vi "ScanDelay_FTIR_PointSpectroscopy.vi"() -> ()   [LabVIEW 2022 SP3] (continued)
  in  "BB-reference spectrum":bool
  in  "Acquire only\nBB 100% curve":bool
  in  "Toggle pause (ms)":dbl=1000.0
  out "BB-referenced spectrum (phase)":T1(graph)
  out "BB-referenced spectrum (amplitude)":T2(graph)
  out "Reference BB spectra":dbl[][](array[numeric])
  out "Reference spectra":dbl[][](array[numeric])
  out "Latest alpha cmd":string="@mir setpump 50.0"
  in  "Replicate\nalpha on\naccumulation":bool=TRUE
  out "# Accumulated":i32=21
  in  "Accumulate to #":i32=21
  in  "Cancel\nacquisition":bool
  out "Toggle position":i32=2
  out "Spectrum stored":bool=TRUE
  out "Reference stored":bool=TRUE
  out "Normalized spectrum (phase)":T1(graph)
  out "Normalized spectrum (amplitude)":T1(graph)
  in  "Store as reference":bool
  out "Python alpha rep path":path=path "C:/Users/mnopl/Desktop/software/mnOPSuite/PRISM/python/alpha.py"
  out "Activity status":string="Awaiting command"
  out "Acquisition status":string="Ready to acquire spectrum"
  in  "Path to save spectrum":path=path "D:/Dropbox/Data/Park-SNOM/2022.07.19 - Liam - Strained STO/11_30 Measurements/Spectra/S2_AuRef12_9.txt"
  in  "Load reference":bool
  in  "Path to load reference":path=path "D:/Dropbox/Data/Park-SNOM/2022.07.19 - Liam - Strained STO/12_7 Measurements/STO_undeformed_S2.txt"
  in  "Path to load spectrum":path=path "D:/Dropbox/Data/Park-SNOM/2022.07.19 - Liam - Strained STO/12_7 Measurements/STO_undeformed_S2.txt"
  in  "Apply spectral\nenvelope":bool=TRUE
  out "Binned interferogram":cluster{"X":dbl, "Y":dbl}[](graph)
  out "Sample BB Spectra":dbl[][](array[numeric])
  out "Sample Spectra":dbl[][](array[numeric])
  out "Python error: spectrum acquisition":errorcluster
  out "Python scandelay path":path=path "C:/Users/mnopl/Desktop/software/mnOPSuite/PRISM/python/scandelay_FTIR.py"
  in  "Time per\nacquisition (s)":dbl=0.18
  in  "Sampling rate":dbl=250000.0
  in  "Delay calibratior\nfactor (ps/V)":dbl=-2.432 format="%_6g"
  in  "Cyc. / intfg.\n(sample)":i32=150
  out "Accumulated spectrum (amplitude)":T3(graph)
  out "Acquisition cycle":dbl[][](graph)
  out "% averaged":dbl=100.0
  in  "Halt program":bool=TRUE
  out "Python error: activity loop":errorcluster
  in  "Load spectrum":bool
  in  "Save spectrum":bool
  in  "Normalize spectrum":bool
  in  "Acquire spectrum":bool
  # "ai6 (7ps): -2 to -5"
  # "ai2 (7ps): -12 to -15"
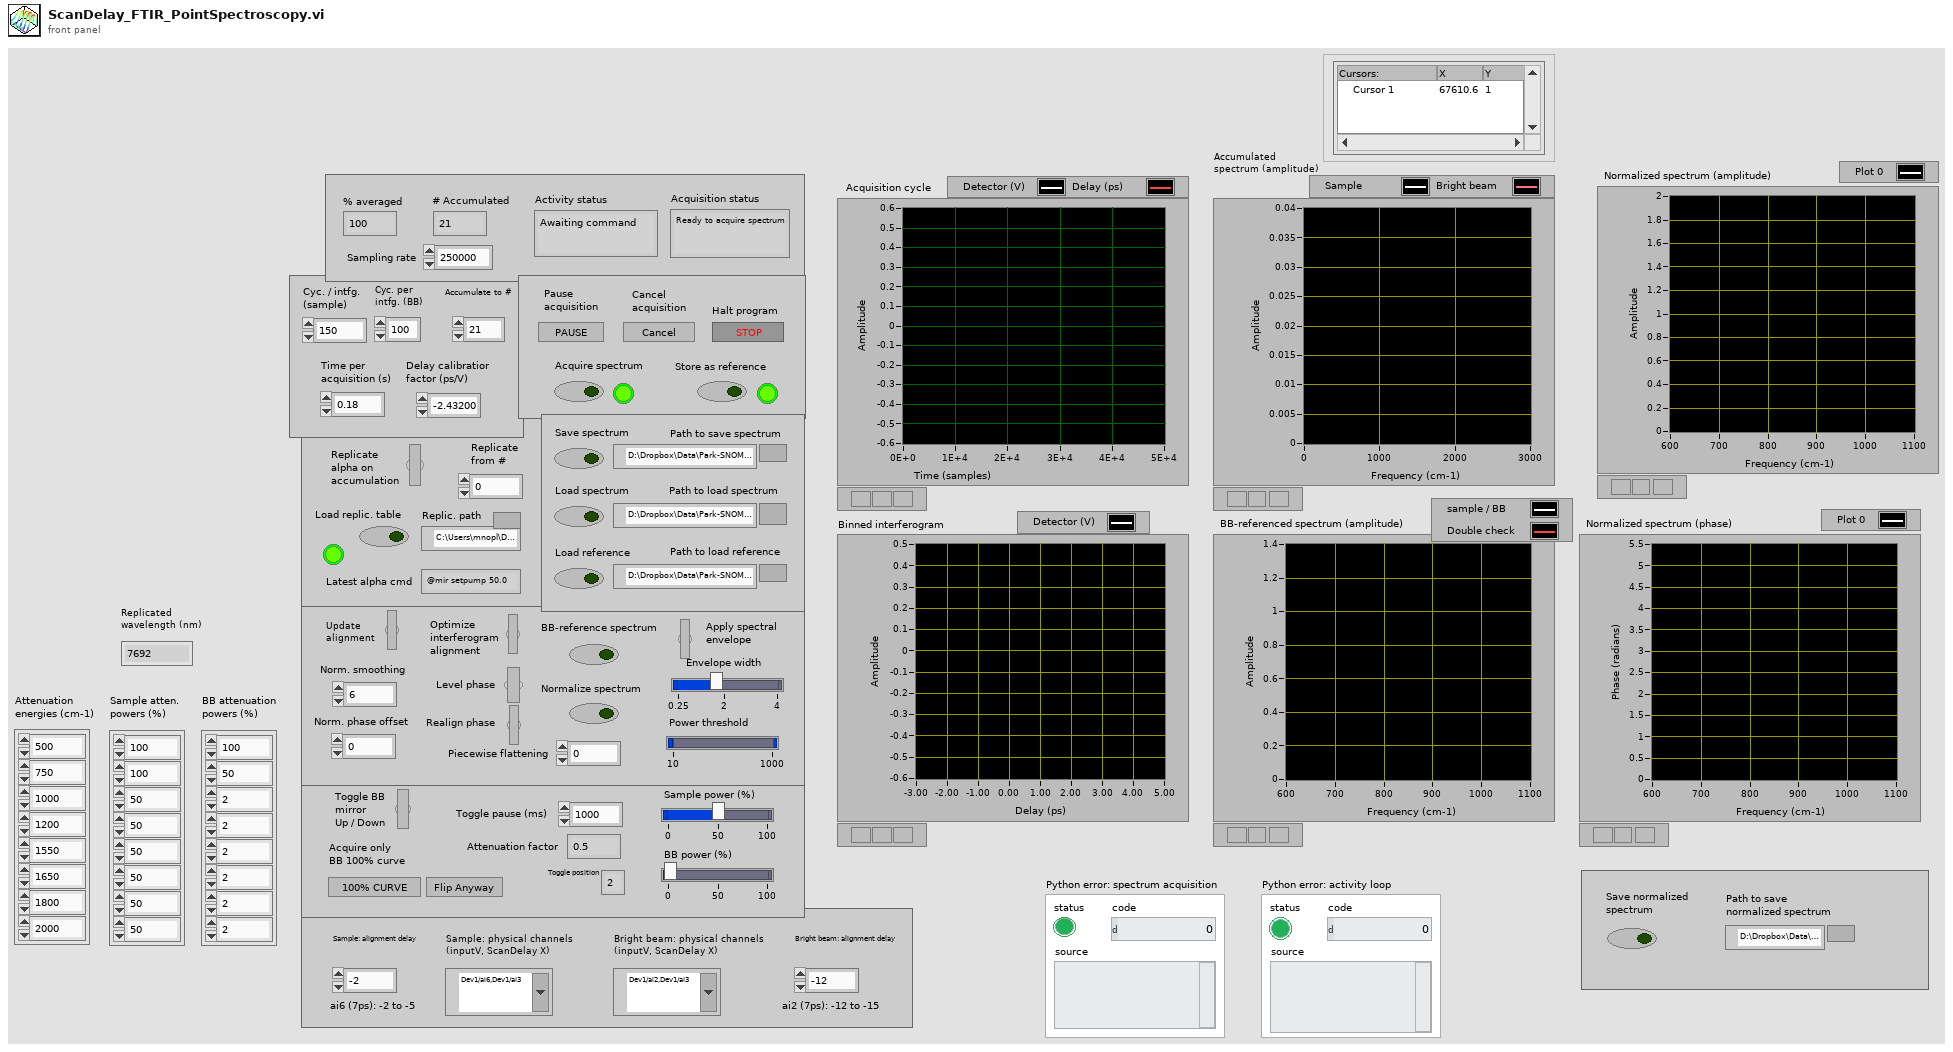
[diagram p1: front panel]
types:
  T1 = cluster{"Output spectrum":dbl[], "Output spectrum":dbl[]}
  T2 = cluster{"Sample Spectra":dbl[], "Sample Spectra":dbl[]}
  T3 = cluster{"Output spectrum":dbl[], "Output spectrum":dbl[]}[]
  T4 = typedef "Control_scanDelayWorkflow.ctl" = enum16{"Hyperspectrum at point", "Sit Idle", "Initialize", "Unpack hyperspectrum", "Slice hyperspectrum", "Linecut norm. at position", "Linecut norm. at frequency", "Next Point", "Load replicator table", "Flip BB", "Load Spectrum", "Store reference", "Save Spectrum", "Load reference", "Check Reference", "Check Spectrum", "Heal linescan", "BB reference spectrum", "BB reference linescan", "Normalize Spectrum", "Normalize Linescan", "Save normalized spectrum", "Save Linescan", "Load Linescan", "Done"}
  T5 = typedef "imagedata.ctl" = cluster{"image type":i32, "image depth":i32, "image":u8[], "mask":u8[], "colors":u32[], "Rectangle":cluster{"left":i16, "top":i16, "right":i16, "bottom":i16}}
  T6 = typedef "Control_GetSpectrum_BBnorm_AttenuateBB.ctl" = enum16{"Initialize", "Replicate alpha", "Flip in BB", "Attenuate alpha", "Get Spectrum", "Accumulate BB spectrum", "Flip out BB", "Accumulate sample spectrum", "Assess accumulation", "Finalize", "Done"}
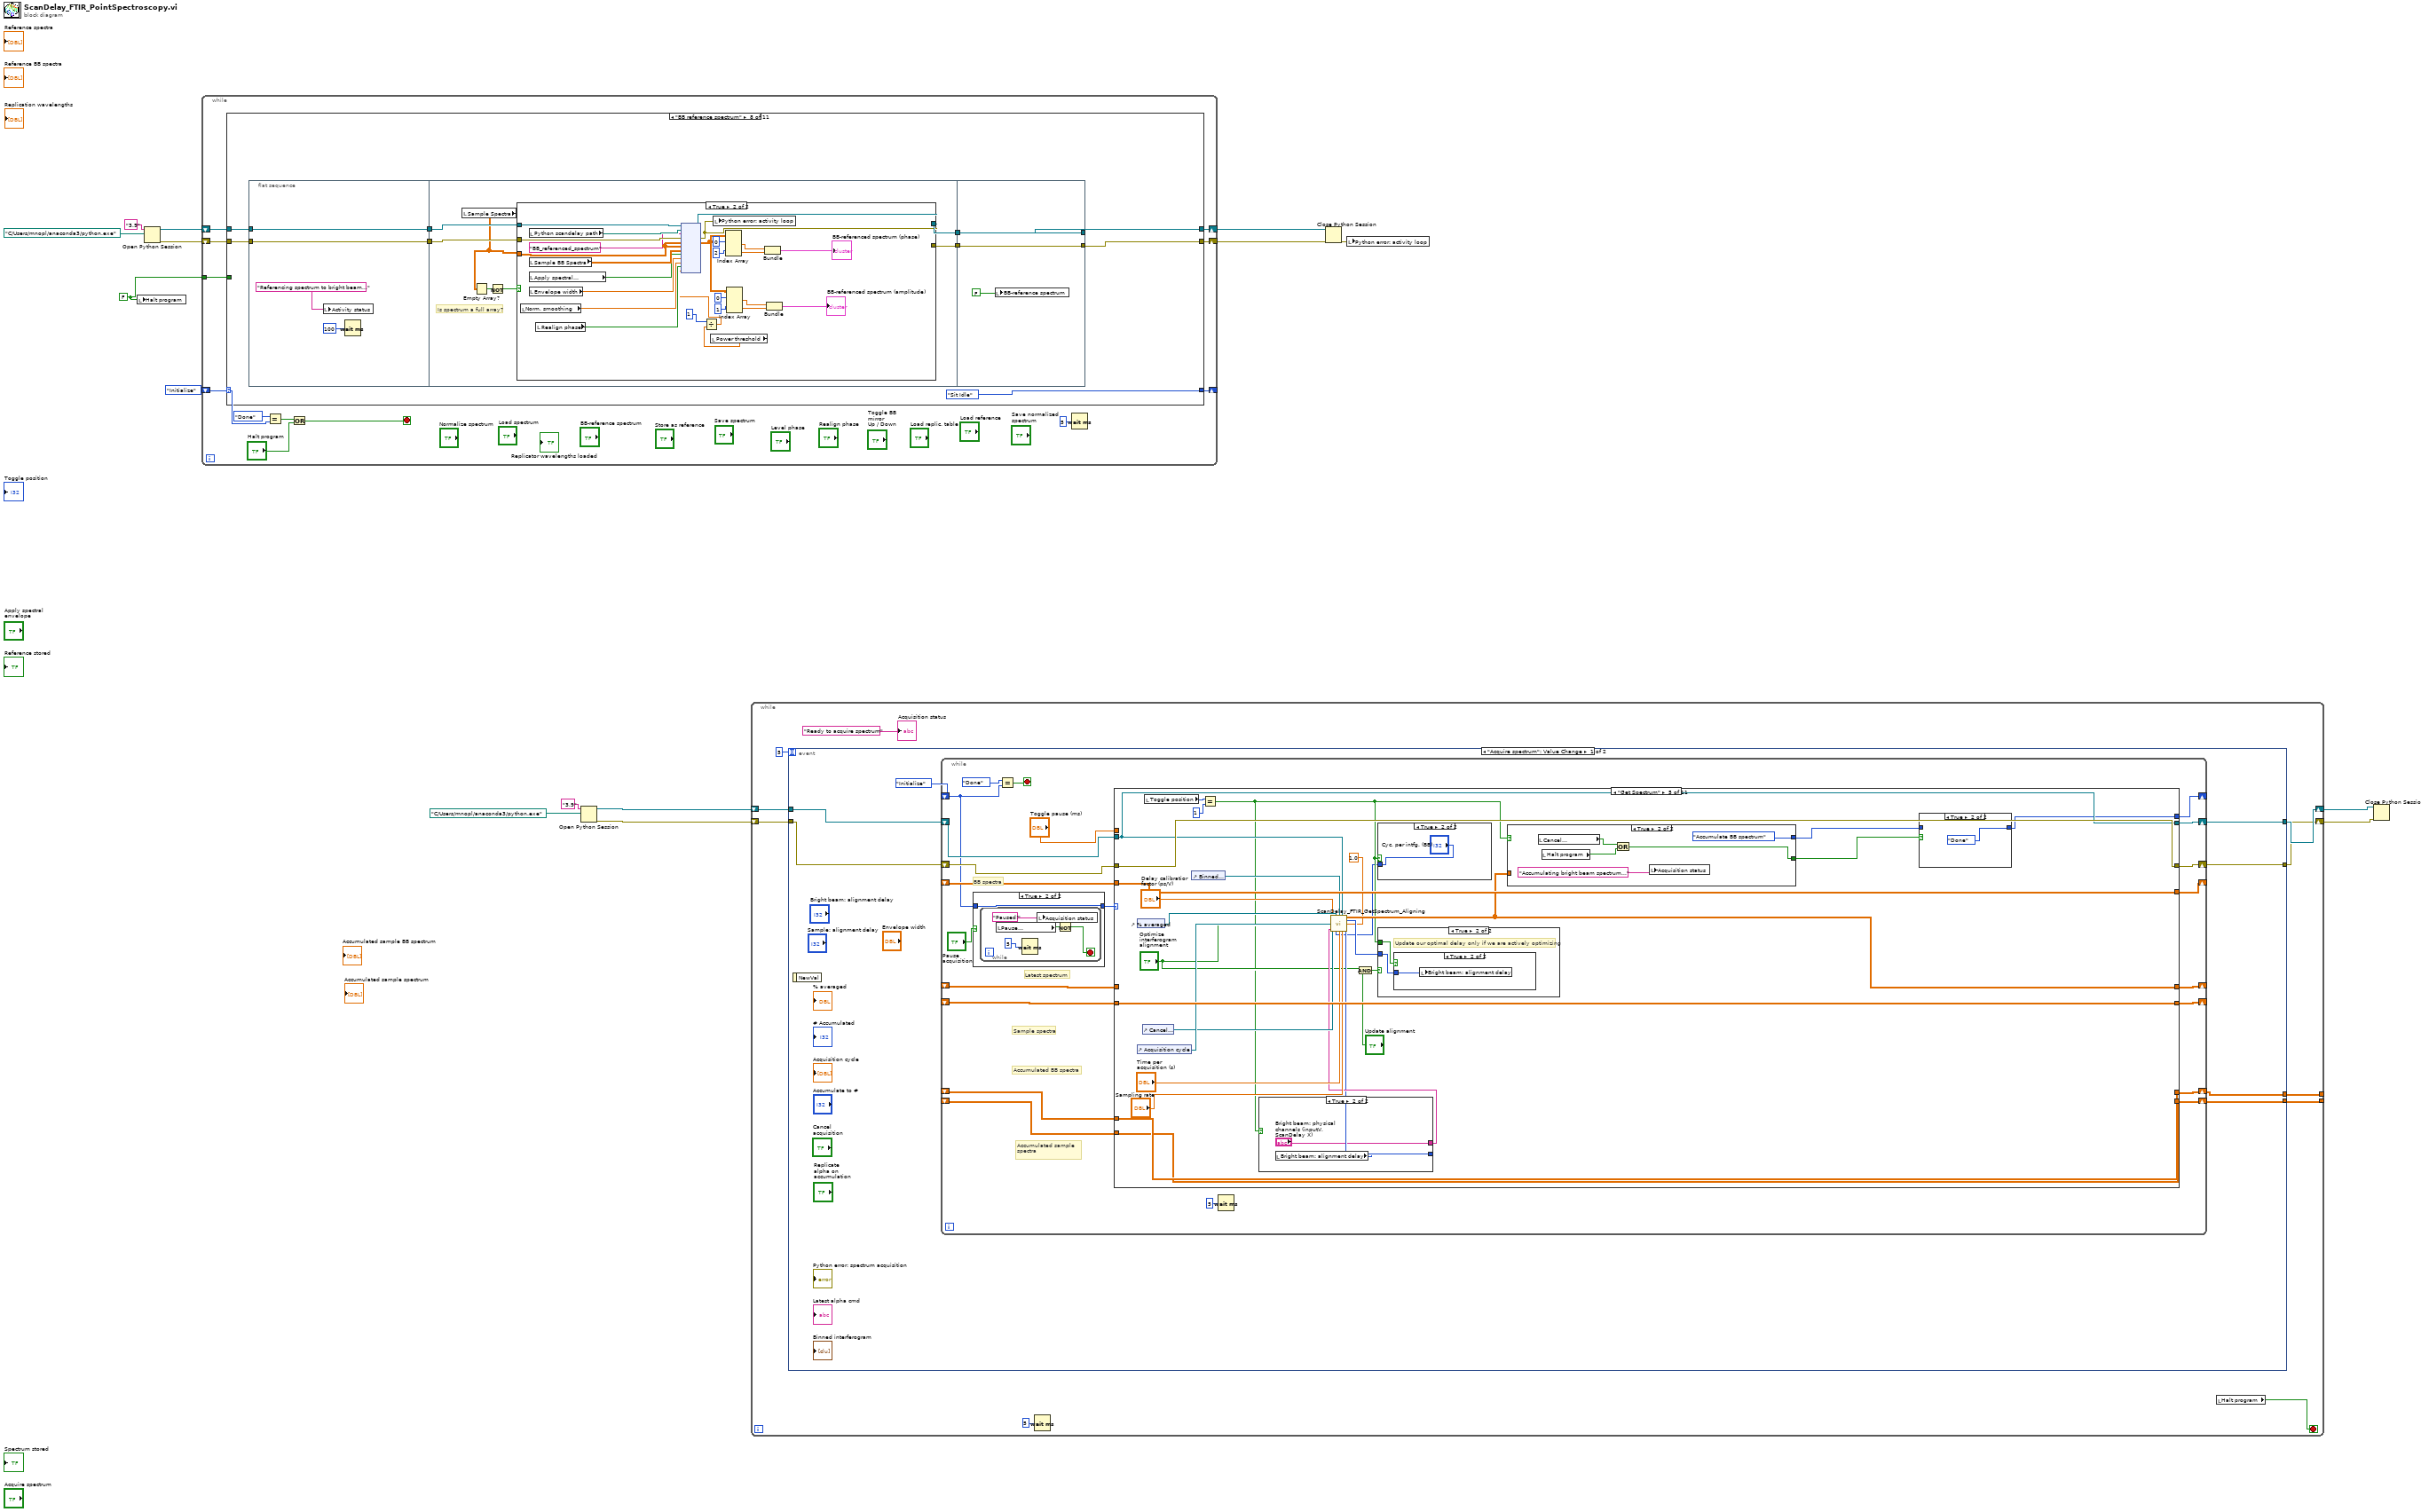
[diagram p0: block diagram]
diagram:
  w1 = FALSE
  n1 = local write "Halt program"(w1) -> ()
  n2 = Open Python Session(python version="3.9", python path=path "C:/Users/mnopl/anaconda3/python.exe") -> (session out=w11:refnum<k35>, error out=w10:errorcluster)  [unwired: 1 in]
  n3 = while {
    shift-right: [w20] -> _
    shift-left: Control_scanDelayWorkflow."Initialize" -> [w17]
    shift-right: [w26] -> w12
    shift-left: w10 -> [w18]
    shift-right: [w21] -> w13
    shift-left: w11 -> [w19]
    tunnel: w1 -> [w16]
    stop <- w24 stop-if-true
    n4 = case shown="\"BB reference spectrum\"" w17 {
      tunnel: [w31 w74 w87 w109 w130 w181 w202 w213 w259 w266 w310] -> w26
      tunnel: w19 -> [w32 w73 w86 w110 w133 w182 w203 w211 w260 w267 w311]
      tunnel: w18 -> [w31 w74 w87 w109 w132 w181 w202 w210 w259 w266 w310]
      tunnel: [w32 w73 w86 w110 w131 w182 w203 w212 w260 w267 w311] -> w21
      tunnel: [w30 Control_scanDelayWorkflow."Sit Idle" Control_scanDelayWorkflow."Sit Idle" Control_scanDelayWorkflow."Sit Idle" Control_scanDelayWorkflow."Sit Idle" Control_scanDelayWorkflow."Sit Idle" Control_scanDelayWorkflow."Sit Idle" Control_scanDelayWorkflow."Sit Idle" Control_scanDelayWorkflow."Sit Idle" Control_scanDelayWorkflow."Sit Idle" Control_scanDelayWorkflow."Sit Idle"] -> w20
      tunnel: w16 -> [_ _ _ _ _ _ w199 _ _ _ _]
      frame "Sit Idle", Default {
        n5 = event shown="[5] \"Load replic. table\": Value Change" {
          selector: _ -> [_ _ _ _ _ _ _ _ _ _]
          dyn-events: _ -> [_ _ _ _ _ _ _ _ _ _]
          timeout: 5 -> [_ _ _ _ _ _ _ _ _ w66]
          tunnel: [w33 w37 w44 Control_scanDelayWorkflow."Flip BB" w46 w50 w54 w58 w62 Control_scanDelayWorkflow."Sit Idle"] -> w30
          event "Normalize spectrum": Value Change {
            n6 = event-data() -> ("NewVal"=w34:bool)  [unwired: 1 in]
            n7 = Select(t=Control_scanDelayWorkflow."Normalize Spectrum", s=w34, f=Control_scanDelayWorkflow."Sit Idle") -> (s? t:f=w33:T4)
          }
          event "Store as reference": Value Change {
            n8 = event-data() -> ("NewVal"=w40:bool)  [unwired: 1 in]
            n9 = Select(t=Control_scanDelayWorkflow."Store reference", s=w40, f=Control_scanDelayWorkflow."Sit Idle") -> (s? t:f=w37:T4)
          }
          event "BB-reference spectrum": Value Change {
            n10 = event-data() -> ("NewVal"=w42:bool)  [unwired: 1 in]
            n11 = Select(t=Control_scanDelayWorkflow."BB reference spectrum", s=w42, f=Control_scanDelayWorkflow."Sit Idle") -> (s? t:f=w44:T4)
          }
          event "Toggle BB\nmirror\nUp / Down": Value Change {
            n12 = event-data() -> ()  [unwired: 1 in, 1 out]
          }
          event "Save normalized\nspectrum": Value Change {
            n13 = event-data() -> ("NewVal"=w47:bool)  [unwired: 1 in]
            n14 = Select(t=Control_scanDelayWorkflow."Save normalized spectrum", s=w47, f=Control_scanDelayWorkflow."Sit Idle") -> (s? t:f=w46:T4)
          }
          event "Load replic. table": Value Change {
            n15 = event-data() -> ("NewVal"=w53:bool)  [unwired: 1 in]
            n16 = Select(t=Control_scanDelayWorkflow."Load replicator table", s=w53, f=Control_scanDelayWorkflow."Sit Idle") -> (s? t:f=w50:T4)
          }
          event "Save spectrum": Value Change {
            n17 = event-data() -> ("NewVal"=w55:bool)  [unwired: 1 in]
            n18 = Select(t=Control_scanDelayWorkflow."Save Spectrum", s=w55, f=Control_scanDelayWorkflow."Sit Idle") -> (s? t:f=w54:T4)
          }
          event "Load reference": Value Change {
            n19 = event-data() -> ("NewVal"=w61:bool)  [unwired: 1 in]
            n20 = Select(t=Control_scanDelayWorkflow."Load reference", s=w61, f=Control_scanDelayWorkflow."Sit Idle") -> (s? t:f=w58:T4)
          }
          event "Load spectrum": Value Change {
            n21 = event-data() -> ("NewVal"=w63:bool)  [unwired: 1 in]
            n22 = Select(t=Control_scanDelayWorkflow."Load Spectrum", s=w63, f=Control_scanDelayWorkflow."Sit Idle") -> (s? t:f=w62:T4)
          }
          event Timeout {
            n23 = event-data() -> ()  [unwired: 1 in, 2 out]
            n24 = Wait (ms)(milliseconds to wait=w66) -> ()  [unwired: 1 out]
          }
        }
        "Activity status" <- "Awaiting command"
      }
      frame "Store reference" {
        # "Is spectrum a full array?"
        n25 = local read "Sample Spectra"() -> (w69:dbl[][])
        n26 = local read "Sample BB Spectra"() -> (w68:dbl[][])
        n27 = Empty Array?(array=w69) -> (empty?=w71:bool)
        n28 = Not(x=w71) -> (.not. x?=w70:bool)
        n29 = case shown="True" w70 {
          tunnel: w69 -> [_ w77]
          tunnel: w68 -> [_ w78]
          frame False {
            n30 = Wait (ms)(milliseconds to wait=1000) -> ()  [unwired: 1 out]
            n31 = local write "Activity status"("Error: Spectrum is empty!") -> ()
          }
          frame True {
            n32 = local write "Reference BB spectra"(w78) -> ()
            n33 = local write "Reference spectra"(w77) -> ()
            n34 = local write "Reference stored"(TRUE) -> ()
            n35 = Wait (ms)(milliseconds to wait=1000) -> ()  [unwired: 1 out]
            n36 = local write "Activity status"("Storing reference!") -> ()
          }
        }
      }
      frame "Save Spectrum" {
        # "Is spectrum a full array?"
        n37 = local read "Sample Spectra"() -> (w83:dbl[][])
        n38 = Empty Array?(array=w83) -> (empty?=w84:bool)
        n39 = Not(x=w84) -> (.not. x?=w82:bool)
        n40 = case shown="False" w82 {
          tunnel: w83 -> [_ w90]
          frame False {
            n41 = flat-sequence {
              frame #0 {
                n42 = local write "Activity status"("Error:  Spectrum is empty, cannot save!") -> ()
              }
              frame #1 {
                n43 = Wait (ms)(milliseconds to wait=1000) -> ()  [unwired: 1 out]
              }
            }
          }
          frame True {
            n44 = flat-sequence {
              tunnel: w90 -> [w91]
              frame #0 {
                w97 = "%g"
                n45 = Path To String(path="Path to save spectrum") -> (string=w100:string)
                n46 = local read "Sample BB Spectra"() -> (w92:dbl[][])
                n47 = Search and Replace String(input string=w100, search string="(.txt)*$", replace string=".txt") -> (result string=w104:string)  [unwired: 5 in, 3 out]
                n48 = Search and Replace String(input string=w104, search string=".txt$", replace string="_BB.txt") -> (result string=w103:string)  [unwired: 5 in, 3 out]
                n49 = String To Path(string=w104) -> (path=w101:path)
                n50 = Array To Spreadsheet String(array=w91, 3:w97) -> (spreadsheet string=w98:string)  [unwired: 1 in]
                n51 = Array To Spreadsheet String(array=w92, 3:w97) -> (spreadsheet string=w105:string)  [unwired: 1 in]
                n52 = String To Path(string=w103) -> (path=w102:path)
                n53 = Write to Text File(file (use dialog)=w101, text=w98) -> ()  [unwired: 2 in, 3 out]
                n54 = Write to Text File(file (use dialog)=w102, text=w105) -> ()  [unwired: 2 in, 3 out]
              }
              frame #1 {
                n55 = local write "Activity status"("Successfully saved spectrum!") -> ()
                n56 = Wait (ms)(milliseconds to wait=1000) -> ()  [unwired: 1 out]
              }
            }
          }
        }
      }
      frame "Load reference" {
        n57 = flat-sequence {
          frame #0 {
            w115 = "%g"
            n58 = Path To String(path="Path to load reference") -> (string=w111:string)
            n59 = Search and Replace String(input string=w111, search string=".txt$", replace string="_BB.txt") -> (result string=w113:string)  [unwired: 5 in, 3 out]
            n60 = Read from Text File(file (use dialog)="Path to load reference") -> (text=w116:string)  [unwired: 3 in, 3 out]
            n61 = String To Path(string=w113) -> (path=w120:path)
            n62 = Spreadsheet String To Array(format string=w115, spreadsheet string=w116) -> (array=w117:dbl[][])  [unwired: 2 in]
            n63 = Read from Text File(file (use dialog)=w120) -> (text=w119:string)  [unwired: 3 in, 3 out]
            n64 = local write "Reference spectra"(w117) -> ()
            n65 = Spreadsheet String To Array(format string=w115, spreadsheet string=w119) -> (array=w121:dbl[][])  [unwired: 2 in]
            n66 = local write "Reference BB spectra"(w121) -> ()
          }
          frame #1 {
            n67 = local write "Reference stored"(TRUE) -> ()
            n68 = Wait (ms)(milliseconds to wait=1000) -> ()  [unwired: 1 out]
            n69 = local write "Activity status"("Successfully loaded reference!") -> ()
          }
        }
      }
      frame "Normalize Spectrum" {
        n70 = local read "Reference stored"() -> (w127:bool)
        n71 = local read "Spectrum stored"() -> (w126:bool)
        n72 = And(x=w126, y=w127) -> (x .and. y?=w125:bool)
        n73 = flat-sequence {
          tunnel: w133 -> [w139]
          tunnel: w132 -> [w138]
          tunnel: [w137] -> w129
          tunnel: [w136] -> w128
          tunnel: w125 -> [w135]
          tunnel: [w178] -> w130
          tunnel: [w179] -> w131
          tunnel: w129 -> [w179]
          tunnel: w128 -> [w178]
          frame #0 {
            n74 = case shown="True" w135 {
              tunnel: w139 -> [w141 w175]
              tunnel: w138 -> [w140 w174]
              tunnel: [w141 w173] -> w137
              tunnel: [w140 w156] -> w136
              frame False {
                n75 = Wait (ms)(milliseconds to wait=1000) -> ()  [unwired: 1 out]
                n76 = local write "Activity status"("Error: Spectrum or reference is empty!") -> ()
              }
              frame True {
                n77 = Wait (ms)(milliseconds to wait=1000) -> ()  [unwired: 1 out]
                n78 = local read "Python scandelay path"() -> (w172:path)
                n79 = local read "Sample Spectra"() -> (w157:dbl[][])
                n80 = local read "Sample BB Spectra"() -> (w158:dbl[][])
                n81 = local read "Reference spectra"() -> (w155:dbl[][])
                n82 = local read "Reference BB spectra"() -> (w154:dbl[][])
                n83 = local read "Apply spectral\nenvelope"() -> (w153:bool)
                n84 = local read "Envelope width"() -> (w152:dbl)
                n85 = local read "Realign phase"() -> (w150:bool)
                n86 = local read "Level phase"() -> (w151:bool)
                n87 = local write "Activity status"("Normalizing spectrum!") -> ()
                n88 = Divide(x=1, y="Power threshold") -> (x/y=w145:dbl)
                n89 = node(w175, w172, "normalized_spectrum", w174, w157, w157, w158, w155, w154, w153, w152, w151, w150, "Norm. phase offset", "Norm. smoothing", w145, "Piecewise flattening") -> (w173:refnum<k35>, w156:errorcluster, w160:dbl[][])  [unwired: 12 in, 2 out]
                "Python error: activity loop" <- w156
                n90 = Index Array(array=w160, index (row) #1=0, index (row) #2=1) -> (element #1=w168:dbl[], element #2=w167:dbl[])  [unwired: 2 in]
                n91 = Index Array(array=w160, index (row) #1=0, index (row) #2=2) -> (element #1=w164:dbl[], element #2=w163:dbl[])  [unwired: 2 in]
                n92 = Bundle("Sample Spectra"=w168, "Sample Spectra"=w167) -> (→"Normalized spectrum (amplitude)":T2)  [unwired: 1 in]
                n93 = Bundle("Sample Spectra"=w164, "Sample Spectra"=w163) -> (→"Normalized spectrum (phase)":T2)  [unwired: 1 in]
              }
            }
          }
          frame #1 {
            n94 = local write "Normalize spectrum"(FALSE) -> ()
          }
        }
      }
      frame "Load Spectrum" {
        n95 = flat-sequence {
          frame #0 {
            w190 = "%g"
            n96 = Path To String(path="Path to load spectrum") -> (string=w186:string)
            n97 = Search and Replace String(input string=w186, search string=".txt$", replace string="_BB.txt") -> (result string=w188:string)  [unwired: 5 in, 3 out]
            n98 = Read from Text File(file (use dialog)="Path to load spectrum") -> (text=w191:string)  [unwired: 3 in, 3 out]
            n99 = String To Path(string=w188) -> (path=w193:path)
            n100 = Spreadsheet String To Array(format string=w190, spreadsheet string=w191) -> (array=w184:dbl[][])  [unwired: 2 in]
            n101 = Read from Text File(file (use dialog)=w193) -> (text=w192:string)  [unwired: 3 in, 3 out]
            n102 = Spreadsheet String To Array(format string=w190, spreadsheet string=w192) -> (array=w183:dbl[][])  [unwired: 2 in]
            n103 = local write "Sample Spectra"(w184) -> ()
            n104 = local write "Sample BB Spectra"(w183) -> ()
          }
          frame #1 {
            n105 = local write "Load spectrum"(FALSE) -> ()
            n106 = local write "Spectrum stored"(TRUE) -> ()
            n107 = local write "Activity status"("Successfully loaded spectrum!") -> ()
            n108 = Wait (ms)(milliseconds to wait=1000) -> ()  [unwired: 1 out]
          }
        }
      }
      frame "Initialize" {
        # "Fine so long as we've saved default values for \"replication wavelengths\""
        n109 = local write "Replicator wavelengths loaded"(TRUE) -> ()
        n110 = local write "Reference stored"(w199) -> ()
        n111 = local write "Spectrum stored"(w199) -> ()
        n112 = local write "Acquire spectrum"(w199) -> ()
        "Python scandelay path" <- path "C:/Users/mnopl/Desktop/software/mnOPSuite/PRISM/python/scandelay_FTIR.py"
        "Python alpha rep path" <- path "C:/Users/mnopl/Desktop/software/mnOPSuite/PRISM/python/alpha.py"
      }
      frame "BB reference spectrum" {
        n113 = flat-sequence {
          tunnel: w210 -> [w216]
          tunnel: w211 -> [w217]
          tunnel: [w217] -> w206
          tunnel: [w216] -> w205
          tunnel: [w224] -> w208
          tunnel: [w223] -> w207
          tunnel: w206 -> [w222]
          tunnel: w205 -> [w221]
          tunnel: [w256] -> w212
          tunnel: [w257] -> w213
          tunnel: w208 -> [w257]
          tunnel: w207 -> [w256]
          frame #0 {
            n114 = local write "Activity status"("Referencing spectrum to bright beam...") -> ()
            n115 = Wait (ms)(milliseconds to wait=100) -> ()  [unwired: 1 out]
          }
          frame #1 {
            # "Is spectrum a full array?"
            n116 = local read "Sample Spectra"() -> (w218:dbl[][])
            n117 = Empty Array?(array=w218) -> (empty?=w220:bool)
            n118 = Not(x=w220) -> (.not. x?=w219:bool)
            n119 = case shown="True" w219 {
              tunnel: [w225 w236] -> w224
              tunnel: [w226 w237] -> w223
              tunnel: w222 -> [w226 w244]
              tunnel: w221 -> [w225 w243]
              tunnel: w218 -> [_ w241]
              frame False {
                n120 = Wait (ms)(milliseconds to wait=500) -> ()  [unwired: 1 out]
                n121 = local write "Activity status"("Error: Spectrum or reference is empty!") -> ()
              }
              frame True {
                n122 = local read "Norm. smoothing"() -> (w229:dbl)
                n123 = local read "Python scandelay path"() -> (w240:path)
                n124 = local read "Sample BB Spectra"() -> (w242:dbl[][])
                n125 = local read "Apply spectral\nenvelope"() -> (w235:bool)
                n126 = local read "Envelope width"() -> (w234:dbl)
                n127 = local read "Realign phase"() -> (w233:bool)
                n128 = local read "Power threshold"() -> (w231:dbl)
                n129 = Divide(x=1, y=w231) -> (x/y=w230:dbl)
                n130 = node(w244, w240, "BB_referenced_spectrum", w243, w241, w241, w242, w235, w234, w229, w233, w230) -> (w237:refnum<k35>, w236:errorcluster, w249:dbl[][])  [unwired: 7 in, 2 out]
                n131 = local write "Python error: activity loop"(w236) -> ()
                n132 = Index Array(array=w249, index (row) #1=0, index (row) #2=2) -> (element #1=w252:dbl[], element #2=w251:dbl[])  [unwired: 2 in]
                n133 = Index Array(array=w249, index (row) #1=0, index (row) #2=1) -> (element #1=w254:dbl[], element #2=w253:dbl[])  [unwired: 2 in]
                n134 = Bundle("Sample Spectra"=w252, "Sample Spectra"=w251) -> (→"BB-referenced spectrum (phase)":T2)  [unwired: 1 in]
                n135 = Bundle("Sample Spectra"=w254, "Sample Spectra"=w253) -> (→"BB-referenced spectrum (amplitude)":T2)  [unwired: 1 in]
              }
            }
          }
          frame #2 {
            n136 = local write "BB-reference spectrum"(FALSE) -> ()
          }
        }
      }
      frame "Flip BB" {
        n137 = local read "Toggle BB\nmirror\nUp / Down"() -> (w262:bool)
        n138 = local read "Toggle pause (ms)"() -> (w258:dbl)
        n139 = call "NewportFlipper.vi"("Settle time (ms)"=w258, "Up/Down"=w262) -> ()  [unwired: 10 in]
      }
      frame "Save normalized spectrum" {
        n140 = flat-sequence {
          tunnel: [w281] -> w268
          tunnel: [w269] -> w263
          tunnel: w268 -> [w295]
          tunnel: [w292] -> w264
          tunnel: w263 -> [w292]
          tunnel: w264 -> [w304]
          frame #0 {
            w286 = "%g"
            n141 = Path To String(path="Path to save\nnormalized spectrum") -> (string=w281:string)
            n142 = property on="Normalized spectrum (phase)" class="XYGraph (strict)"() -> ("Value"=w271:T1)  [unwired: 2 in, 2 out]
            n143 = property on="Normalized spectrum (amplitude)" class="XYGraph (strict)"() -> ("Value"=w279:T1)  [unwired: 2 in, 2 out]
            n144 = Unbundle(w279) -> ("Output spectrum"=w278:dbl[], "Output spectrum"=w277:dbl[])
            n145 = Unbundle(w271) -> ("Output spectrum"=w274:dbl[], "Output spectrum"=w273:dbl[])
            n146 = Build Array(w278, w277) -> (w276:dbl[][])
            n147 = Build Array(w274, w273) -> (w272:dbl[][])
            n148 = Search and Replace String(input string=w281, search string="(.txt)$", replace string="_normalized_phase.txt") -> (result string=w290:string)  [unwired: 5 in, 3 out]
            n149 = Search and Replace String(input string=w281, search string="(.txt)*$", replace string="_normalized_amplitude.txt") -> (result string=w269:string)  [unwired: 5 in, 3 out]
            n150 = Transpose 2D Array(2D array=w276) -> (transposed array=w275:dbl[][])
            n151 = Transpose 2D Array(2D array=w272) -> (transposed array=w270:dbl[][])
            n152 = Array To Spreadsheet String(array=w275, 3:w286) -> (spreadsheet string=w291:string)  [unwired: 1 in]
            n153 = Array To Spreadsheet String(array=w270, 3:w286) -> (spreadsheet string=w287:string)  [unwired: 1 in]
            n154 = String To Path(string=w290) -> (path=w289:path)
            n155 = String To Path(string=w269) -> (path=w288:path)
            n156 = Write to Text File(file (use dialog)=w289, text=w291) -> ()  [unwired: 2 in, 3 out]
            n157 = Write to Text File(file (use dialog)=w288, text=w287) -> ()  [unwired: 2 in, 3 out]
          }
          frame #1 {
            n158 = invoke on="Normalized spectrum (amplitude)" class="XYGraph (strict)" method="Get Image"() -> ("image data"=w294:T5)  [unwired: 6 in, 5 out]
            n159 = Search and Replace String(input string=w295, search string="(.txt)$", replace string="_normalized_amplitude.png") -> (result string=w301:string)  [unwired: 5 in, 3 out]
            n160 = String To Path(string=w301) -> (path=w300:path)
            n161 = call <vilib>:"Write PNG File.vi"("image data"=w294, "path to PNG file"=w300) -> ()  [unwired: 8 in, 2 out]
            n162 = invoke on="Normalized spectrum (phase)" class="XYGraph (strict)" method="Get Image"() -> ("image data"=w293:T5)  [unwired: 6 in, 5 out]
            n163 = Search and Replace String(input string=w295, search string="(.txt)$", replace string="_normalized_phase.png") -> (result string=w297:string)  [unwired: 5 in, 3 out]
            n164 = String To Path(string=w297) -> (path=w296:path)
            n165 = call <vilib>:"Write PNG File.vi"("image data"=w293, "path to PNG file"=w296) -> ()  [unwired: 8 in, 2 out]
          }
          frame #2 {
            n166 = local write "Save normalized\nspectrum"(FALSE) -> ()
            n167 = Concatenate Strings("Spectrum successfully saved to:" ("message"), "\r", w304) -> (w307:string)
            n168 = One Button Dialog(message=w307, button name ("OK")="OK") -> ()  [unwired: 1 out]
          }
        }
      }
      frame "Load replicator table" {
        n169 = flat-sequence {
          frame #0 {
            # "A leading whitespace in replication table requires skipping an extra column"
            n170 = Read from Text File(file (use dialog)="Replic. path") -> (text=w319:string)  [unwired: 3 in, 3 out]
            n171 = Spreadsheet String To Array(delimiter (Tab)=" ", format string="%g", spreadsheet string=w319) -> (array=w316:dbl[][])  [unwired: 1 in]
            n172 = Index Array(array=w316, index (col)=4) -> (element=w314:dbl[])  [unwired: 1 in]
            n173 = local write "Replication wavelengths"(w314) -> ()
          }
          frame #1 {
            n174 = local write "Load replic. table"(FALSE) -> ()
            n175 = local write "Replicator wavelengths loaded"(TRUE) -> ()
            n176 = Wait (ms)(milliseconds to wait=1000) -> ()  [unwired: 1 out]
            n177 = local write "Activity status"("Successfully loaded replication wavelengths!") -> ()
          }
        }
      }
    }
    n178 = Equal?(x=Control_scanDelayWorkflow."Done", y=w17) -> (x = y?=w22:bool)
    n179 = Or(x=w22, y="Halt program") -> (x .or. y?=w24:bool)
    n180 = Wait (ms)(milliseconds to wait=5) -> ()  [unwired: 1 out]
  }
  n181 = Open Python Session(python version="3.9", python path=path "C:/Users/mnopl/anaconda3/python.exe") -> (session out=w5:refnum<k35>, error out=w4:errorcluster)  [unwired: 1 in]
  n182 = while {
    shift-right: [w326] -> w2
    shift-left: w4 -> [w328]
    shift-right: [w327] -> w3
    shift-left: w5 -> [w329]
    tunnel: [w325] -> _
    tunnel: [w324] -> _
    stop <- w333 stop-if-true
    n183 = event shown="[0] \"Acquire spectrum\": Value Change" {
      selector: _ -> [_ _]
      dyn-events: _ -> [_ _]
      timeout: 5 -> [_ w665]
      tunnel: w329 -> [w339 w664]
      tunnel: w328 -> [w338 w663]
      tunnel: [w337 w664] -> w327
      tunnel: [w336 w663] -> w326
      tunnel: [w335 _] -> w325
      tunnel: [w334 _] -> w324
      event "Acquire spectrum": Value Change {
        n184 = event-data() -> ()  [unwired: 1 in, 1 out]
        n185 = while {
          shift-right: [w360] -> _
          shift-left: _ -> [w359]
          shift-right: [w361] -> _
          shift-left: _ -> [w358]
          shift-right: [w357] -> _
          shift-left: Control_GetSpectrum_BBnorm_AttenuateBB."Initialize" -> [w343]
          shift-right: [w354] -> w336
          shift-left: w338 -> [w355]
          shift-right: [w353] -> w337
          shift-left: w339 -> [w356]
          shift-right: [w352] -> _
          shift-left: _ -> [w350]
          shift-right: [w348] -> w335
          shift-left: _ -> [w346]
          shift-right: [w347] -> w334
          shift-left: _ -> [w345]
          stop <- w342 stop-if-true
          # "BB spectra"
          # "Accumulated BB spectra"
          # "Accumulated sample spectra"
          # "Sample spectra"
          # "Latest spectrum"
          n186 = case shown="True" "Pause\nacquisition" {
            tunnel: w343 -> [w363 w364]
            tunnel: [w363 w364] -> w341
            frame False {
            }
            frame True {
              n187 = while {
                stop <- w368 stop-if-true
                n188 = local read "Pause\nacquisition"() -> (w367:bool)
                n189 = Wait (ms)(milliseconds to wait=5) -> ()  [unwired: 1 out]
                n190 = local write "Acquisition status"("Paused!") -> ()
                n191 = Not(x=w367) -> (.not. x?=w368:bool)
              }
            }
          }
          n192 = Equal?(x=Control_GetSpectrum_BBnorm_AttenuateBB."Done", y=w343) -> (x = y?=w342:bool)
          n193 = case shown="\"Get Spectrum\"" w341 {
            tunnel: [w369 w399 w407 w445 w500 w537 w571 w598 w620 w647 w658] -> w361
            tunnel: [w369 w400 w408 w443 w499 w548 w572 w591 w621 w646 w660] -> w360
            tunnel: w359 -> [_ w400 w408 w443 w499 w557 w572 w591 w621 w646 w660]
            tunnel: w358 -> [_ w399 w407 w445 w500 w537 w571 w599 w620 w647 w658]
            tunnel: [w375 Control_GetSpectrum_BBnorm_AttenuateBB."Flip in BB" Control_GetSpectrum_BBnorm_AttenuateBB."Attenuate alpha" w419 w484 w528 Control_GetSpectrum_BBnorm_AttenuateBB."Attenuate alpha" Control_GetSpectrum_BBnorm_AttenuateBB."Assess accumulation" w623 Control_GetSpectrum_BBnorm_AttenuateBB."Done" Control_GetSpectrum_BBnorm_AttenuateBB."Done"] -> w357